vi "UHR-Fleezers Control (host) - 12.8.1.vi"() -> ()   [LabVIEW 2012] (continued)
          tunnel: ["W/ Offset 1"] -> w675
          tunnel: w678 -> [w724]
          tunnel: w675 -> [w722]
          frame #0 {
            n416 = property on="Sample Channel\nFlow" class="Bool (strict)"("Val(Sgnl)"="Daq spot flow on") -> ()  [unwired: 2 in, 2 out]
            n417 = Wait (ms)(milliseconds to wait=u32 250) -> ()  [unwired: 1 out]
          }
          frame #1 {
            n418 = local read "Saved Stage Positions"() -> (w687:dbl[][])
            n419 = property on="Trap Delta (MHz)" class="DigNum (strict)"("Val(Sgnl)"="Cal @ (MHz)") -> ()  [unwired: 2 in, 2 out]
            n420 = local write "Stage Moving"(TRUE ("Stage Moving")) -> ()
            n421 = call "move to saved stage position.vi"("error in"=w689, "Stage VISA resource name in"=w690, "Position"="Cal Stage Position", "Saved Stage Positions"=w687) -> ("error out"=w688:errorcluster)  [unwired: 1 out]
            n422 = local write "Stage Control Serial Error"(w688) -> ()
          }
          frame #2 {
            n423 = local write "Stage Moving"(FALSE ("Stage Moving")) -> ()
            n424 = property on="Sample Channel\nFlow" class="Bool (strict)"("Val(Sgnl)"="Flow ON during cal?") -> ()  [unwired: 2 in, 2 out]
            n425 = call <vilib>:"Beep.vi"() -> ()  [unwired: 3 in, 9 out]
          }
          frame #3 {
            n426 = Wait (ms)(milliseconds to wait=u32 1000) -> ()  [unwired: 1 out]
          }
          frame #4 {
            n427 = property on="Save Calibration" class="Bool (strict)"("Val(Sgnl)"=TRUE ("Value (Signaling)")) -> ()  [unwired: 2 in, 2 out]
          }
          frame #5 {
            n428 = Wait (ms)(milliseconds to wait=u32 2000) -> ()  [unwired: 1 out]
          }
          frame #6 {
            # "Check to see if \nsaving done"
            n429 = while {
              stop <- w699 stop-if-true
              n430 = local read "Saving..."() -> (w700:bool)
              n431 = Wait (ms)(milliseconds to wait=u32 100) -> ()  [unwired: 1 out]
              n432 = Not(x=w700) -> (.not. x?=w699:bool)
            }
          }
          frame #7 {
            n433 = case shown="True" "W/ Offset 1" {
              tunnel: w703 -> [_ w704]
              frame False {
              }
              frame True {
                n434 = stacked-sequence {
                  tunnel: w704 -> [_ _ _ _ _ _ _ w721]
                  frame #0 {
                    n435 = property on="Trap Delta (MHz)" class="DigNum (strict)"("Val(Sgnl)"="Offset 1 Start (MHz)") -> ()  [unwired: 2 in, 2 out]
                    n436 = Replace Array Subset(array=u32[] [0] ("Index Values"), new element="Offset 1 Set", index=0) -> (w705:u32[])
                    n437 = property on="Saved AOD Raster Scan Parameter Sets" class="Arr (strict)"("Index Values"=w705) -> ()  [unwired: 2 in, 2 out]
                  }
                  frame #1 {
                    n438 = Wait (ms)(milliseconds to wait=u32 200) -> ()  [unwired: 1 out]
                  }
                  frame #2 {
                    n439 = property on="Load parameters" class="Bool (strict)"("Val(Sgnl)"=TRUE ("Value (Signaling)")) -> ()  [unwired: 2 in, 2 out]
                  }
                  frame #3 {
                    n440 = Wait (ms)(milliseconds to wait=u32 200) -> ()  [unwired: 1 out]
                  }
                  frame #4 {
                    n441 = property on="Trap Raster Scan" class="Bool (strict)"("Val(Sgnl)"=TRUE ("Value (Signaling)")) -> ()  [unwired: 2 in, 2 out]
                  }
                  frame #5 {
                    n442 = Wait (ms)(milliseconds to wait=u32 2000) -> ()  [unwired: 1 out]
                  }
                  frame #6 {
                    n443 = while {
                      stop <- w718 stop-if-true
                      n444 = local read "Raster Scanning..."() -> (w720:bool)
                      n445 = local read "Saving..."() -> (w716:bool)
                      n446 = Wait (ms)(milliseconds to wait=u32 100) -> ()  [unwired: 1 out]
                      n447 = Not(x=w716) -> (.not. x?=w715:bool)
                      n448 = Not(x=w720) -> (.not. x?=w717:bool)
                      n449 = And(x=w717, y=w715) -> (x .and. y?=w718:bool)
                    }
                  }
                  frame #7 {
                    n450 = property on="Trap Delta (MHz)" class="DigNum (strict)"("Val(Sgnl)"=w721) -> ()  [unwired: 2 in, 2 out]
                  }
                }
              }
            }
          }
          frame #8 {
            n451 = local read "Save ave N"() -> (w723:dbl)
            n452 = case shown="False" "W/ Offset 2" {
              tunnel: w724 -> [_ w731]
              tunnel: w723 -> [_ w730]
              tunnel: w722 -> [w726 _]
              frame False {
                n453 = case shown="False" w726 {
                  frame False {
                    n454 = Multiply(x="Cal read wait (s)", y=u32 1000 ("milliseconds to wait")) -> (x*y=w728:u32)
                    n455 = Wait (ms)(milliseconds to wait=w728) -> ()  [unwired: 1 out]
                  }
                  frame True {
                  }
                }
              }
              frame True {
                n456 = stacked-sequence {
                  tunnel: w731 -> [_ _ _ _ _ _ _ _ _ w752 _ _]
                  tunnel: w730 -> [_ _ _ _ _ _ _ _ _ w750 _ _]
                  frame #0 {
                    n457 = property on="Save ave N" class="DigNum (strict)"("Val(Sgnl)"=1.0 ("Value (Signaling)")) -> ()  [unwired: 2 in, 2 out]
                  }
                  frame #1 {
                    n458 = Wait (ms)(milliseconds to wait=u32 500) -> ()  [unwired: 1 out]
                  }
                  frame #2 {
                    n459 = property on="Trap Delta (MHz)" class="DigNum (strict)"("Val(Sgnl)"="Offset 2 Start (MHz)") -> ()  [unwired: 2 in, 2 out]
                    n460 = Replace Array Subset(array=u32[] [0] ("Index Values"), new element="Offset 2 Set", index=0) -> (w736:u32[])
                    n461 = property on="Saved AOD Raster Scan Parameter Sets" class="Arr (strict)"("Index Values"=w736) -> ()  [unwired: 2 in, 2 out]
                  }
                  frame #3 {
                    n462 = Wait (ms)(milliseconds to wait=u32 500) -> ()  [unwired: 1 out]
                  }
                  frame #4 {
                    n463 = property on="Load parameters" class="Bool (strict)"("Val(Sgnl)"=TRUE ("Value (Signaling)")) -> ()  [unwired: 2 in, 2 out]
                  }
                  frame #5 {
                    n464 = Wait (ms)(milliseconds to wait=u32 500) -> ()  [unwired: 1 out]
                  }
                  frame #6 {
                    n465 = property on="Trap Raster Scan" class="Bool (strict)"("Val(Sgnl)"=TRUE ("Value (Signaling)")) -> ()  [unwired: 2 in, 2 out]
                  }
                  frame #7 {
                    n466 = Wait (ms)(milliseconds to wait=u32 2000) -> ()  [unwired: 1 out]
                  }
                  frame #8 {
                    n467 = while {
                      stop <- w745 stop-if-true
                      n468 = local read "Raster Scanning..."() -> (w748:bool)
                      n469 = local read "Saving..."() -> (w746:bool)
                      n470 = Wait (ms)(milliseconds to wait=u32 100) -> ()  [unwired: 1 out]
                      n471 = Not(x=w746) -> (.not. x?=w744:bool)
                      n472 = Not(x=w748) -> (.not. x?=w747:bool)
                      n473 = And(x=w747, y=w744) -> (x .and. y?=w745:bool)
                    }
                  }
                  frame #9 {
                    n474 = property on="Trap Delta (MHz)" class="DigNum (strict)"("Val(Sgnl)"=w752) -> ()  [unwired: 2 in, 2 out]
                    n475 = property on="Saved AOD Raster Scan Parameter Sets" class="Arr (strict)"("Index Values"=u32[] [0]) -> ()  [unwired: 2 in, 2 out]
                    n476 = property on="Save ave N" class="DigNum (strict)"("Val(Sgnl)"=w750) -> ()  [unwired: 2 in, 2 out]
                  }
                  frame #10 {
                    n477 = Wait (ms)(milliseconds to wait=u32 500) -> ()  [unwired: 1 out]
                  }
                  frame #11 {
                    n478 = property on="Load parameters" class="Bool (strict)"("Val(Sgnl)"=TRUE ("Value (Signaling)")) -> ()  [unwired: 2 in, 2 out]
                  }
                }
              }
            }
          }
          frame #9 {
            n479 = property on="Read Cal" class="Bool (strict)"("Val(Sgnl)"=TRUE ("Value (Signaling)")) -> ()  [unwired: 2 in, 2 out]
          }
          frame #10 {
            n480 = Wait (ms)(milliseconds to wait=u32 1000) -> ()  [unwired: 1 out]
          }
          frame #11 {
            n481 = property on="Fish for Tether" class="Bool (strict)"("Val(Sgnl)"=TRUE ("Value (Signaling)")) -> ()  [unwired: 2 in, 2 out]
          }
        }
        n482 = local write "Cal/Data Acq. Spot"(FALSE ("Cal/Data Acq. Spot")) -> ()
      }
      event "Dump Beads": Value Change {
        n483 = event-data() -> ()  [unwired: 1 in, 5 out]
        n484 = flat-sequence {
          tunnel: ["Dump spot flow on?"] -> w758
          tunnel: [w769] -> w759
          tunnel: w758 -> [w769]
          tunnel: w762 -> [w774]
          tunnel: w761 -> [w773]
          tunnel: [w771] -> w760
          tunnel: w759 -> [w771]
          tunnel: w760 -> [w784]
          frame #0 {
            w763 = FALSE ("Value (Signaling)")
            n485 = local read "Saving..."() -> (w765:bool)
            n486 = local write "Dump Beads"(FALSE ("Dump Beads")) -> ()
            n487 = property on="Inject Pump 3" class="Bool (strict)"("Val(Sgnl)"=w763) -> ()  [unwired: 2 in, 2 out]
            n488 = property on="Inject Pump 1" class="Bool (strict)"("Val(Sgnl)"=w763) -> ()  [unwired: 2 in, 2 out]
            n489 = local write "Stop Saving"(w765) -> ()
          }
          frame #1 {
            w766 = FALSE ("Fl. Triggered...")
            n490 = case shown="True" "Dump spot flow on?" {
              frame False {
              }
              frame True {
                n491 = property on="Sample Channel\nFlow" class="Bool (strict)"("Val(Sgnl)"=TRUE ("Stage Moving")) -> ()  [unwired: 2 in, 2 out]
              }
            }
            n492 = local write "Fl. Triggered..."(w766) -> ()
            n493 = local write "Tether"(w766) -> ()
            n494 = property on="Green Laser ON" class="Bool (strict)"("Val(Sgnl)"=w766) -> ()  [unwired: 2 in, 2 out]
            n495 = property on="Trap Pos. FB ON" class="Bool (strict)"("Val(Sgnl)"=w766) -> ()  [unwired: 2 in, 2 out]
            n496 = property on="Trap Trig. Fl." class="Bool (strict)"("Val(Sgnl)"=w766) -> ()  [unwired: 2 in, 2 out]
            n497 = property on="Fl. Triggered..." class="Bool (strict)"("Val(Sgnl)"=w766) -> ()  [unwired: 2 in, 2 out]
            n498 = property on="Dip for Protein" class="Bool (strict)"("Val(Sgnl)"=w766) -> ()  [unwired: 2 in, 2 out]
            n499 = property on="Pause dwell" class="Bool (strict)"("Val(Sgnl)"=w766) -> ()  [unwired: 2 in, 2 out]
          }
          frame #2 {
            n500 = property on="Trap Pos. FB Offset Factor" class="DigNum (strict)"("Val(Sgnl)"=i64 0 ("Value (Signaling)")) -> ()  [unwired: 2 in, 2 out]
          }
          frame #3 {
            n501 = local read "Saved Stage Positions"() -> (w775:dbl[][])
            n502 = local write "Stage Moving"(TRUE ("Stage Moving")) -> ()
            n503 = Array Subset(array=w775, index (row)=3 ("index"), length (row)=1 ("length"), index (col)=1 ("index"), length (col)=3 ("length")) -> (w780:dbl[][])
            n504 = Reshape Array(w780, 3 ("dimension size")) -> (w778:dbl[])
            n505 = Array To Cluster(array=w778) -> (cluster=w777:cluster{"[0]":dbl, "[1]":dbl, "[2]":dbl})
            n506 = call "Set Stage Position.vi"("Position"=w777, "error in"=w773, "VISA resource name in"=w774) -> ()  [unwired: 3 out]
          }
          frame #4 {
            w785 = FALSE ("Value (Signaling)")
            n507 = case shown="True" w784 {
              frame False {
              }
              frame True {
                n508 = property on="Sample Channel\nFlow" class="Bool (strict)"("Val(Sgnl)"=FALSE ("Stage Moving")) -> ()  [unwired: 2 in, 2 out]
              }
            }
            n509 = property on="Trap 1 (ON/OFF)" class="Bool (strict)"("Val(Sgnl)"=w785) -> ()  [unwired: 2 in, 2 out]
            n510 = property on="Trap 2 (ON/OFF)" class="Bool (strict)"("Val(Sgnl)"=w785) -> ()  [unwired: 2 in, 2 out]
            n511 = call <vilib>:"Beep.vi"() -> ()  [unwired: 3 in, 9 out]
          }
          frame #5 {
            n512 = property on="Move Cap. 2 (ADig Top)" class="Bool (strict)"("Val(Sgnl)"=TRUE ("Value (Signaling)")) -> ()  [unwired: 2 in, 2 out]
            n513 = property on="Tab Control" class="TabCtl (strict)"("Val(Sgnl)"=T30."Status" ("Value (Signaling)")) -> ()  [unwired: 2 in, 2 out]
          }
        }
      }
      event "Dip for Protein": Value Change {
        n514 = event-data() -> ()  [unwired: 1 in, 5 out]
        n515 = case shown="True" "Dip for Protein" {
          tunnel: w791 -> [_ w793]
          tunnel: w790 -> [_ w792]
          frame False {
          }
          frame True {
            n516 = while {
              tunnel: w793 -> [w804]
              tunnel: w792 -> [w803]
              i -> [w798]
              stop <- w800 stop-if-true
              n517 = Increment(x=w798) -> (x+1=→"Dip #":i32)
              n518 = flat-sequence {
                tunnel: w803 -> [w815]
                tunnel: w804 -> [w816]
                tunnel: [w816] -> w808
                tunnel: [w815] -> w807
                tunnel: [w809] -> w794
                tunnel: [w821] -> w802
                tunnel: [w822] -> w801
                tunnel: w808 -> [w823]
                tunnel: w807 -> [w824]
                tunnel: [w819] -> w795
                tunnel: w794 -> [w819]
                tunnel: [w832] -> w806
                tunnel: w802 -> [w832]
                tunnel: [w831] -> w805
                tunnel: w801 -> [w831]
                tunnel: [w828] -> w799
                tunnel: [w827] -> w796
                tunnel: w795 -> [w827]
                tunnel: w805 -> [w852]
                tunnel: w806 -> [w853]
                tunnel: w799 -> [w854]
                tunnel: w796 -> [w851]
                tunnel: [w910] -> w800
                frame #0 {
                  n519 = local read "Trap Pos. FB ON"() -> (w809:bool)
                  n520 = Compound Arithmetic op=AND("Flow ON\nduring dip?", "FB OFF when \nflow ON", w809) -> (w810:bool)
                  n521 = case shown="True" "Move trap \nbefore dip move?" {
                    frame False {
                    }
                    frame True {
                      n522 = property on="Trap Delta (MHz)" class="DigNum (strict)"("Val(Sgnl)"="Dipping Delta (MHz)") -> ()  [unwired: 2 in, 2 out]
                    }
                  }
                  n523 = property on="Green Laser ON" class="Bool (strict)"("Val(Sgnl)"="Green ON\nbefore dip?") -> ()  [unwired: 2 in, 2 out]
                  n524 = property on="Sample Channel\nFlow" class="Bool (strict)"("Val(Sgnl)"="Flow ON\nduring dip?") -> ()  [unwired: 2 in, 2 out]
                  n525 = case shown="True" w810 {
                    frame False {
                    }
                    frame True {
                      n526 = property on="Trap Pos. FB ON" class="Bool (strict)"("Val(Sgnl)"=FALSE ("Value (Signaling)")) -> ()  [unwired: 2 in, 2 out]
                    }
                  }
                }
                frame #1 {
                  n527 = local read "Saved Stage Positions"() -> (w826:dbl[][])
                  n528 = local write "Cancel dwell"(FALSE ("Cancel dwell")) -> ()
                  n529 = call "move to saved stage position.vi"("error in"=w824, "Stage VISA resource name in"=w823, "Position"="Dip Stage \nPosition", "Saved Stage Positions"=w826) -> ("VISA resource name out"=w821:refnum<visa-resource-name>, "error out"=w822:errorcluster)
                }
                frame #2 {
                  n530 = node-c288() -> (w830:T27)  [unwired: 4 in]
                  n531 = timed-loop {
                    timing: w830 -> [_]
                    timing-out: [_] -> w829
                    tunnel: [w836] -> w828
                    i -> [w833]
                    stop <- w837 stop-if-true
                    n532 = node-c288() -> ()  [unwired: 1 in, 1 out]
                    n533 = Greater Or Equal?(x=w833, y="Dip Duration (s)") -> (x >= y?=w845:bool)
                    n534 = local read "Dip for Protein"() -> (w838:bool)
                    n535 = local read "Dump Beads"() -> (w835:bool)
                    n536 = local read "Cancel dwell"() -> (w844:bool)
                    n537 = local read "Pause dwell"() -> (w841:bool)
                    n538 = Not(x=w838) -> (.not. x?=w843:bool)
                    n539 = Compound Arithmetic op=OR(w844, w845, w843) -> (w842:bool)
                    n540 = Select(t=FALSE, s=w841, f=w842) -> (s? t:f=w839:bool)
                    n541 = Not(x=w835) -> (.not. x?=w834:bool)
                    n542 = node-c288() -> ()  [unwired: 1 in, 1 out]
                    n543 = And(x=w838, y=w834) -> (x .and. y?=w836:bool)
                    n544 = Or(x=w839, y=w835) -> (x .or. y?=w837:bool)
                    "Dip Time (s)" <- w833
                  }
                  n545 = node-c288(w829) -> ()  [unwired: 1 out]
                }
                frame #3 {
                  n546 = case shown="True" w854 {
                    tunnel: w853 -> [_ w859]
                    tunnel: w852 -> [_ w858]
                    tunnel: w851 -> [_ w855]
                    frame False {
                    }
                    frame True {
                      n547 = flat-sequence {
                        tunnel: w858 -> [w863]
                        tunnel: w859 -> [w864]
                        tunnel: [w864] -> w857
                        tunnel: [w863] -> w856
                        tunnel: w855 -> [w860]
                        tunnel: w857 -> [w874]
                        tunnel: w856 -> [w873]
                        tunnel: w855 -> [w882]
                        frame #0 {
                          n548 = local read "Sample Channel\nFlow"() -> (w862:bool)
                          n549 = case shown="True" w862 {
                            tunnel: "Flow ON \nduring return\nfrom dip?" -> [w865 w868]
                            tunnel: w860 -> [_ w867]
                            frame False {
                              n550 = case shown="True" w865 {
                                frame False {
                                }
                                frame True {
                                n551 = property on="Sample Channel\nFlow" class="Bool (strict)"("Val(Sgnl)"=TRUE ("Value (Signaling)")) -> ()  [unwired: 2 in, 2 out]
                                }
                              }
                            }
                            frame True {
                              n552 = case shown="False" w868 {
                                tunnel: w867 -> [w869 _]
                                frame False {
                                n553 = property on="Trap Pos. FB ON" class="Bool (strict)"("Val(Sgnl)"=w869) -> ()  [unwired: 2 in, 2 out]
                                n554 = property on="Sample Channel\nFlow" class="Bool (strict)"("Val(Sgnl)"=FALSE ("Value (Signaling)")) -> ()  [unwired: 2 in, 2 out]
                                }
                                frame True {
                                }
                              }
                            }
                          }
                        }
                        frame #1 {
                          # "For turning on green laser before stage reaches lower spot"
                          n555 = case shown="True" "Green ON\nafter start\nreturn?" {
                            frame False {
                            }
                            frame True {
                              n556 = flat-sequence {
                                frame #0 {
                                n557 = Multiply(x="Green delay after \nstart return (s)", y=1000.0) -> (x*y=w879:dbl)
                                n558 = Wait (ms)(milliseconds to wait=w879) -> ()  [unwired: 1 out]
                                }
                                frame #1 {
                                n559 = property on="Green Laser ON" class="Bool (strict)"("Val(Sgnl)"=TRUE ("Value (Signaling)")) -> ()  [unwired: 2 in, 2 out]
                                }
                              }
                            }
                          }
                          n560 = local read "Saved Stage Positions"() -> (w877:dbl[][])
                          n561 = local write "Cancel dwell"(FALSE ("Cancel dwell")) -> ()
                          n562 = call "move to saved stage position.vi"("error in"=w873, "Stage VISA resource name in"=w874, "Position"="Return Stage \nPosition", "Saved Stage Positions"=w877) -> ("error out"=w875:errorcluster)  [unwired: 1 out]
                          n563 = local write "Stage Control Serial Error"(w875) -> ()
                        }
                        frame #2 {
                          n564 = property on="Trap Pos. FB ON" class="Bool (strict)"("Val(Sgnl)"=w882) -> ()  [unwired: 2 in, 2 out]
                          n565 = case shown="True" "Green ON \nafter return?" {
                            frame False {
                            }
                            frame True {
                              n566 = property on="Green Laser ON" class="Bool (strict)"("Val(Sgnl)"=TRUE ("Value (Signaling)")) -> ()  [unwired: 2 in, 2 out]
                            }
                          }
                          n567 = case shown="True" "Move trap after return?" {
                            frame False {
                            }
                            frame True {
                              n568 = property on="Trap Delta (MHz)" class="DigNum (strict)"("Val(Sgnl)"="Dip Trap Delta 2 (MHz)") -> ()  [unwired: 2 in, 2 out]
                            }
                          }
                          n569 = case shown="True" "Save data after return?" {
                            frame False {
                            }
                            frame True {
                              n570 = property on="Start Saving" class="Bool (strict)"("Val(Sgnl)"=TRUE ("Value (Signaling)")) -> ()  [unwired: 2 in, 2 out]
                            }
                          }
                          n571 = property on="Sample Channel\nFlow" class="Bool (strict)"("Val(Sgnl)"="Flow ON\nduring daq?") -> ()  [unwired: 2 in, 2 out]
                        }
                        frame #3 {
                          n572 = node-c288() -> (w891:T27)  [unwired: 4 in]
                          n573 = timed-loop {
                            timing: w891 -> [_]
                            timing-out: [_] -> w890
                            i -> [w892]
                            stop <- w894 stop-if-true
                            n574 = node-c288() -> ()  [unwired: 1 in, 1 out]
                            n575 = local read "Dump Beads"() -> (w893:bool)
                            n576 = Greater Or Equal?(x=w892, y="Dwell Duration (s)") -> (x >= y?=w899:bool)
                            n577 = local read "Dip for Protein"() -> (w896:bool)
                            n578 = Not(x=w896) -> (.not. x?=w895:bool)
                            n579 = Compound Arithmetic op=OR(w899, "Cancel dwell", w895) -> (w898:bool)
                            n580 = node-c288() -> ()  [unwired: 1 in, 1 out]
                            n581 = Select(t=FALSE, s="Pause dwell", f=w898) -> (s? t:f=w901:bool)
                            n582 = Or(x=w901, y=w893) -> (x .or. y?=w894:bool)
                            "Dwell Time (s)" <- w892
                          }
                          n583 = node-c288(w890) -> ()  [unwired: 1 out]
                        }
                      }
                    }
                  }
                }
                frame #4 {
                  n584 = local read "Dip for Protein"() -> (w911:bool)
                  n585 = local read "Dump Beads"() -> (w908:bool)
                  n586 = local write "Cancel dwell"(FALSE ("Cancel dwell")) -> ()
                  n587 = Not(x=w911) -> (.not. x?=w912:bool)
                  n588 = Not(x="Cont. Repeat Dipping?") -> (.not. x?=w914:bool)
                  n589 = Compound Arithmetic op=OR(w912, w914, w908) -> (w910:bool)
                }
              }
            }
          }
        }
      }
      event "Profile": Value Change {
        n590 = event-data() -> ()  [unwired: 1 in, 5 out]
        n591 = flat-sequence {
          tunnel: w923 -> [w926]
          tunnel: w922 -> [w934]
          tunnel: [w928] -> w921
          tunnel: [w927] -> w920
          tunnel: [w925] -> w918
          tunnel: [w924] -> w915
          tunnel: w921 -> [w941]
          tunnel: w920 -> [w940]
          tunnel: [w938] -> w919
          tunnel: w918 -> [w939]
          tunnel: [w937] -> w917
          tunnel: [w936] -> w916
          tunnel: w915 -> [w936]
          tunnel: w919 -> [w945]
          tunnel: w917 -> [w944]
          tunnel: w916 -> [w943]
          frame #0 {
            n592 = call "Read Stage Position.vi"("error in"=w934, "VISA resource name in"=w926) -> ("Current Position"=w924:cluster{dbl, dbl, dbl}, "error out"=w927:errorcluster, "VISA resource name out"=w925:refnum<visa-resource-name>)  [unwired: 1 out]
            "Current Position" <- w924
            n593 = local write "Stage Control Serial Error"(w927) -> ()
            n594 = Unbundle(w924) -> (w931:dbl, w933:dbl, w929:dbl)
            n595 = Add(x=w933, y="Y change (mm)") -> (x+y=w930:dbl)
            n596 = Bundle(w931, w930, w929) -> (w928:cluster{dbl, dbl, dbl})  [unwired: 1 in]
          }
          frame #1 {
            # "move to new position and start saving"
            n597 = local write "Stage Moving"(TRUE ("Stage Moving")) -> ()
            n598 = local write "Start Saving"(TRUE ("Start Saving")) -> ()
            n599 = call "Set Stage Position.vi"("Position"=w941, "error in"=w940, "VISA resource name in"=w939) -> ("error out"=w937:errorcluster, "VISA resource name out"=w938:refnum<visa-resource-name>)  [unwired: 1 out]
          }
          frame #2 {
            # "go back to start"
            n600 = call "Set Stage Position.vi"("Position"=w943, "error in"=w944, "VISA resource name in"=w945) -> ()  [unwired: 3 out]
          }
          frame #3 {
            # "stop saving"
            n601 = local write "Stop Saving"(TRUE ("Stop Saving")) -> ()
            n602 = local write "Stage Moving"(FALSE ("Stage Moving")) -> ()
          }
        }
      }
      event "Move to Position 1", "Move to Position 2", "Move to Position 3", "Move to Position 4", "Move to Position 5", "Lower Ch. Cap.": Value Change {
        n603 = event-data() -> ()  [unwired: 1 in, 5 out]
        n604 = Or(x="Move to Position 5", y="Lower Ch. Cap.") -> (x .or. y?=w951:bool)
        n605 = Build Array("Move to Position 1", "Move to Position 2", "Move to Position 3", "Move to Position 4", w951) -> (w954:bool[])
        n606 = Boolean Array To Number(Boolean array=w954) -> (number=w953:u32)
        n607 = Logarithm Base 2(1:w953) -> (0:w952:dbl)
        n608 = flat-sequence {
          tunnel: w952 -> [w963]
          tunnel: w949 -> [w961]
          tunnel: w948 -> [w960]
          frame #0 {
            n609 = local read "Saved Stage Positions"() -> (w971:dbl[][])
            n610 = Array Subset(array=w971, index (row)=w963, length (row)=1 ("length"), index (col)=1 ("index"), length (col)=3 ("length")) -> (w968:dbl[][])
            n611 = Reshape Array(w968, 3 ("dimension size")) -> (w966:dbl[])
            n612 = Array To Cluster(array=w966) -> (cluster=w965:cluster{"[0]":dbl, "[1]":dbl, "[2]":dbl})
            n613 = call "Set Stage Position.vi"("Position"=w965, "error in"=w960, "VISA resource name in"=w961) -> ("error out"=w964:errorcluster)  [unwired: 2 out]
            n614 = local write "Stage Moving"(TRUE ("Stage Moving")) -> ()
            n615 = local write "Stage Control Serial Error"(w964) -> ()
          }
          frame #1 {
            n616 = local write "Stage Moving"(FALSE ("Stage Moving")) -> ()
            n617 = call <vilib>:"Beep.vi"() -> ()  [unwired: 3 in, 9 out]
          }
        }
      }
      event "Got ADig bead": Value Change {
        n618 = event-data() -> ()  [unwired: 1 in, 5 out]
        n619 = flat-sequence {
          frame #0 {
            n620 = local read "Cap 1 Samp Flow ON"() -> (w975:bool)
            n621 = case shown="True" w975 {
              frame False {
              }
              frame True {
                n622 = property on="Sample Channel\nFlow" class="Bool (strict)"("Val(Sgnl)"=TRUE ("Value (Signaling)")) -> ()  [unwired: 2 in, 2 out]
              }
            }
          }
          frame #1 {
            n623 = property on="Inject Pump 3" class="Bool (strict)"("Val(Sgnl)"=FALSE ("Value (Signaling)")) -> ()  [unwired: 2 in, 2 out]
          }
          frame #2 {
            n624 = property on="Move Cap. 1 (DNA Bottom)" class="Bool (strict)"("Val(Sgnl)"=TRUE ("Value (Signaling)")) -> ()  [unwired: 2 in, 2 out]
          }
        }
      }
      event "Force FB Data\nScript": Value Change {
        n625 = event-data() -> ()  [unwired: 1 in, 5 out]
        n626 = flat-sequence {
          tunnel: w984 -> [w988]
          tunnel: w985 -> [w989]
          tunnel: [w989] -> w980
          tunnel: [w988] -> w979
          tunnel: w980 -> [w992]
          tunnel: w979 -> [w991]
          tunnel: ["Trap Trig Fl."] -> w981
          tunnel: [w1017] -> w982
          tunnel: w981 -> [w1017]
          tunnel: [w1021] -> w983
          tunnel: w982 -> [w1021]
          tunnel: w983 -> [w1023]
          frame #0 {
            n627 = property on="Trap Delta (MHz)" class="DigNum (strict)"("Val(Sgnl)"="Trap Delta Before Moving") -> ()  [unwired: 2 in, 2 out]
          }
          frame #1 {
            n628 = local read "Saved Stage Positions"() -> (w994:dbl[][])
            n629 = local write "FB Trap Pos Offset"(0.0 ("FB Trap Pos Offset")) -> ()
            n630 = property on="Trap Pos. FB Offset Factor" class="DigNum (strict)"("Val(Sgnl)"=i64 0 ("Value (Signaling)")) -> ()  [unwired: 2 in, 2 out]
            n631 = local write "Stage Moving"(TRUE ("Stage Moving")) -> ()
            n632 = call "move to saved stage position.vi"("error in"=w991, "Stage VISA resource name in"=w992, "Position"="Stage Position To Establish FB", "Saved Stage Positions"=w994) -> ("error out"=w990:errorcluster)  [unwired: 1 out]
            n633 = local write "Stage Control Serial Error"(w990) -> ()
          }
          frame #2 {
            n634 = call <vilib>:"Beep.vi"() -> ()  [unwired: 3 in, 9 out]
            n635 = Multiply(x="Wait (s)", y=u32 1000 ("milliseconds to wait")) -> (x*y=w1001:u32)
            n636 = property on="Trap Delta (MHz)" class="DigNum (strict)"("Val(Sgnl)"="Starting \nTrap Delta (MHz)") -> ()  [unwired: 2 in, 2 out]
            n637 = local write "Stage Moving"(FALSE ("Stage Moving")) -> ()
            n638 = Wait (ms)(milliseconds to wait=w1001) -> ()  [unwired: 1 out]
            n639 = property on="Tab Control 2" class="TabCtl (strict)"("Val(Sgnl)"=T8."Feedback on Trap Position" ("Value (Signaling)")) -> ()  [unwired: 2 in, 2 out]
            n640 = property on="Tab Control" class="TabCtl (strict)"("Val(Sgnl)"=T31."Trap Control (RF)" ("Value (Signaling)")) -> ()  [unwired: 2 in, 2 out]
          }
          frame #3 {
            n641 = property on="Set Reading to\nSetpoint" class="Bool (strict)"("Val(Sgnl)"=TRUE ("Value (Signaling)")) -> ()  [unwired: 2 in, 2 out]
            n642 = Wait (ms)(milliseconds to wait=u32 500) -> ()  [unwired: 1 out]
          }
          frame #4 {
            n643 = property on="Trap Pos. FB ON" class="Bool (strict)"("Val(Sgnl)"=TRUE ("Value (Signaling)")) -> ()  [unwired: 2 in, 2 out]
            n644 = Wait (ms)(milliseconds to wait=u32 250) -> ()  [unwired: 1 out]
          }
          frame #5 {
            n645 = case shown="False" "Trap Trig Fl." {
              frame False {
                n646 = case shown="True" "Green ON after FB ON?" {
                  selector: "Green ON after FB ON?" -> [_ w1016]
                  frame False {
                  }
                  frame True {
                    n647 = property on="Green Laser ON" class="Bool (strict)"("Val(Sgnl)"=w1016) -> ()  [unwired: 2 in, 2 out]
                  }
                }
              }
              frame True {
              }
            }
            n648 = case shown="True" "Remove Action Offset" {
              tunnel: TRUE ("Value (Signaling)") -> [w1013 w1014]
              frame False {
                n649 = property on="Remove Unwinding Offset" class="Bool (strict)"("Val(Sgnl)"=w1013) -> ()  [unwired: 2 in, 2 out]
              }
              frame True {
                n650 = property on="Remove Action Offset" class="Bool (strict)"("Val(Sgnl)"=w1014) -> ()  [unwired: 2 in, 2 out]
              }
            }
            n651 = Wait (ms)(milliseconds to wait=u32 250) -> ()  [unwired: 1 out]
          }
          frame #6 {
            n652 = property on="Start Saving" class="Bool (strict)"("Val(Sgnl)"=TRUE ("Value (Signaling)")) -> ()  [unwired: 2 in, 2 out]
            n653 = Wait (ms)(milliseconds to wait=u32 5000) -> ()  [unwired: 1 out]
          }
          frame #7 {
            w1020 = TRUE ("Value (Signaling)")
            n654 = property on="Rem fb disp offset" class="Bool (strict)"("Val(Sgnl)"=w1020) -> ()  [unwired: 2 in, 2 out]
            n655 = property on="Remove Offset" class="Bool (strict)"("Val(Sgnl)"=w1020) -> ()  [unwired: 2 in, 2 out]
            n656 = Wait (ms)(milliseconds to wait=u32 100) -> ()  [unwired: 1 out]
          }
          frame #8 {
            n657 = case shown="True" w1023 {
              frame False {
              }
              frame True {
                n658 = local write "Trap Trig. Fl."(TRUE ("Value (Signaling)")) -> ()
              }
            }
          }
          frame #9 {
            n659 = case shown="True" "Start dipping after?" {
              frame False {
              }
              frame True {
                n660 = flat-sequence {
                  frame #0 {
                    n661 = Multiply(x="Delay before dipping (s)", y=1000.0) -> (x*y=w1027:dbl)
                    n662 = Wait (ms)(milliseconds to wait=w1027) -> ()  [unwired: 1 out]
                  }
                  frame #1 {
                    n663 = property on="Dip for Protein" class="Bool (strict)"("Val(Sgnl)"=TRUE ("Value (Signaling)")) -> ()  [unwired: 2 in, 2 out]
                    n664 = local write "Scripts"(T1."Dipping" ("Scripts")) -> ()
                  }
                }
              }
            }
          }
        }
      }
      event "Fixed Traps Data\nScript": Value Change {
        n665 = event-data() -> ()  [unwired: 1 in, 5 out]
        n666 = flat-sequence {
          frame #0 {
            n667 = case shown="True" "Green ON" {
              frame False {
              }
              frame True {
                n668 = property on="Green Laser ON" class="Bool (strict)"("Val(Sgnl)"=TRUE) -> ()  [unwired: 2 in, 2 out]
              }
            }
            n669 = local write "Offset (nm)"(0.0 ("Offset (nm)")) -> ()
            n670 = property on="Sample Channel\nFlow" class="Bool (strict)"("Val(Sgnl)"=FALSE ("Value (Signaling)")) -> ()  [unwired: 2 in, 2 out]
            n671 = property on="Trap Delta (MHz)" class="DigNum (strict)"("Val(Sgnl)"="Fixed Traps Trap Delta (MHz)") -> ()  [unwired: 2 in, 2 out]
          }
          frame #1 {
            n672 = Wait (ms)(milliseconds to wait=u32 1000) -> ()  [unwired: 1 out]
          }
          frame #2 {
            n673 = local write "Start Saving"(TRUE ("Start Saving")) -> ()
          }
          frame #3 {
            n674 = local read "Bead Sep. Int. Time (s)"() -> (w1038:dbl)
            n675 = Multiply(x=w1038, y=1000.0) -> (x*y=w1040:dbl)
            n676 = Wait (ms)(milliseconds to wait=w1040) -> ()  [unwired: 1 out]
          }
          frame #4 {
            n677 = property on="Remove Offset" class="Bool (strict)"("Val(Sgnl)"=TRUE ("Value (Signaling)")) -> ()  [unwired: 2 in, 2 out]
          }
          frame #5 {
            n678 = property on="Dip for Protein" class="Bool (strict)"("Val(Sgnl)"="Start dipping after?") -> ()  [unwired: 2 in, 2 out]
          }
        }
      }
      event "Got DNA bead": Value Change {
        n679 = event-data() -> ()  [unwired: 1 in, 5 out]
        n680 = flat-sequence {
          frame #0 {
            n681 = local read "Daq spot flow on"() -> (w1045:bool)
            n682 = case shown="True" w1045 {
              frame False {
              }
              frame True {
                n683 = property on="Sample Channel\nFlow" class="Bool (strict)"("Val(Sgnl)"=TRUE ("Value (Signaling)")) -> ()  [unwired: 2 in, 2 out]
              }
            }
            n684 = property on="Got DNA bead" class="Bool"("Key Focus"=FALSE) -> ()  [unwired: 2 in, 2 out]
          }
          frame #1 {
            n685 = property on="Inject Pump 1" class="Bool (strict)"("Val(Sgnl)"=FALSE ("Value (Signaling)")) -> ()  [unwired: 2 in, 2 out]
          }
          frame #2 {
            n686 = property on="Cal/Data Acq. Spot" class="Bool (strict)"("Val(Sgnl)"=TRUE ("Value (Signaling)")) -> ()  [unwired: 2 in, 2 out]
          }
        }
      }
      event "Take Stepping Data": Value Change {
        n687 = event-data() -> ()  [unwired: 1 in, 5 out]
        n688 = local read "Save ave N"() -> (w1057:dbl)
        n689 = flat-sequence {
          tunnel: w1057 -> [w1059]
          tunnel: [w1059] -> w1052
          tunnel: [w1061] -> w1053
          tunnel: w1052 -> [w1061]
          tunnel: [w1063] -> w1054
          tunnel: w1053 -> [w1063]
          tunnel: [w1066] -> w1055
          tunnel: w1054 -> [w1066]
          tunnel: [w1068] -> w1056
          tunnel: w1055 -> [w1068]
          tunnel: [w1070] -> w1050
          tunnel: w1056 -> [w1070]
          tunnel: w1050 -> [w1073]
          tunnel: [w1073] -> w1049
          tunnel: w1049 -> [w1074]
          tunnel: [w1074] -> w1051
          tunnel: w1051 -> [w1080]
          frame #0 {
            n690 = property on="Save ave N" class="DigNum (strict)"("Val(Sgnl)"="Save ave factor") -> ()  [unwired: 2 in, 2 out]
          }
          frame #1 {
            n691 = Wait (ms)(milliseconds to wait=u32 100) -> ()  [unwired: 1 out]
          }
          frame #2 {
            n692 = local read "Offset 2 Start (MHz)"() -> (w1065:dbl)
            n693 = property on="Saved AOD Raster Scan Parameter Sets" class="Arr (strict)"("Index Values"=u32[] [2]) -> ()  [unwired: 2 in, 2 out]
            n694 = property on="Trap Delta (MHz)" class="DigNum (strict)"("Val(Sgnl)"=w1065) -> ()  [unwired: 2 in, 2 out]
          }
          frame #3 {
            n695 = property on="Load parameters" class="Bool (strict)"("Val(Sgnl)"=TRUE ("Value (Signaling)")) -> ()  [unwired: 2 in, 2 out]
          }
          frame #4 {
            n696 = Wait (ms)(milliseconds to wait=u32 100) -> ()  [unwired: 1 out]
          }
          frame #5 {
            n697 = property on="Trap Raster Scan" class="Bool (strict)"("Val(Sgnl)"=TRUE ("Value (Signaling)")) -> ()  [unwired: 2 in, 2 out]
          }
          frame #6 {
            n698 = Wait (ms)(milliseconds to wait=u32 1000) -> ()  [unwired: 1 out]
          }
          frame #7 {
            n699 = while {
              stop <- w1077 stop-if-true
              n700 = local read "Raster Scanning..."() -> (w1079:bool)
              n701 = local read "Saving..."() -> (w1078:bool)
              n702 = Not(x=w1078) -> (.not. x?=w1075:bool)
              n703 = Not(x=w1079) -> (.not. x?=w1076:bool)
              n704 = And(x=w1076, y=w1075) -> (x .and. y?=w1077:bool)
            }
          }
          frame #8 {
            n705 = property on="Save ave N" class="DigNum (strict)"("Val(Sgnl)"=w1080) -> ()  [unwired: 2 in, 2 out]
          }
        }
      }
      event "Step Size (nm)": Value Change {
        n706 = event-data() -> ()  [unwired: 1 in, 5 out]
        n707 = flat-sequence {
          frame #0 {
            n708 = property on="Saved AOD Raster Scan Parameter Sets" class="Arr (strict)"("Index Values"=u32[] [1]) -> ()  [unwired: 2 in, 2 out]
          }
          frame #1 {
            n709 = Multiply(x="N Steps", y="Step Size (nm)") -> (x*y=w1082:dbl)
            n710 = property on="Scan Speed AOD (nm/s) 2" class="DigNum (strict)"("Value"="Step Size (nm)") -> ()  [unwired: 2 in, 2 out]
            n711 = property on="Step Size AOD (nm) 2" class="DigNum (strict)"("Value"="Step Size (nm)") -> ()  [unwired: 2 in, 2 out]
            n712 = property on="Scan Range AOD (nm) 2" class="DigNum (strict)"("Value"=w1082) -> ()  [unwired: 2 in, 2 out]
          }
        }
      }
      event "Take Detection Laser\nImage": Value Change {
        n713 = event-data() -> ()  [unwired: 1 in, 5 out]
        n714 = flat-sequence {
          tunnel: [w1110] -> w1100
          tunnel: [w1109] -> w1093
          tunnel: [w1108] -> w1085
          tunnel: [w1113] -> w1101
          tunnel: w1100 -> [w1113]
          tunnel: [w1112] -> w1094
          tunnel: w1093 -> [w1112]
          tunnel: [w1111] -> w1086
          tunnel: w1085 -> [w1111]
          tunnel: [w1117] -> w1102
          tunnel: w1101 -> [w1117]
          tunnel: [w1116] -> w1095
          tunnel: w1094 -> [w1116]
          tunnel: [w1115] -> w1087
          tunnel: w1086 -> [w1115]
          tunnel: [w1123] -> w1103
          tunnel: w1102 -> [w1123]
          tunnel: [w1122] -> w1096
          tunnel: w1095 -> [w1122]
          tunnel: [w1121] -> w1088
          tunnel: w1087 -> [w1121]
          tunnel: [w1127] -> w1104
          tunnel: w1103 -> [w1127]
          tunnel: [w1126] -> w1097
          tunnel: w1096 -> [w1126]
          tunnel: [w1125] -> w1089
          tunnel: w1088 -> [w1125]
          tunnel: [w1131] -> w1105
          tunnel: w1104 -> [w1131]
          tunnel: [w1130] -> w1098
          tunnel: w1097 -> [w1130]
          tunnel: [w1129] -> w1090
          tunnel: w1089 -> [w1129]
          tunnel: [w1135] -> w1106
          tunnel: w1105 -> [w1135]
          tunnel: [w1134] -> w1099
          tunnel: w1098 -> [w1134]
          tunnel: [w1133] -> w1091
          tunnel: w1090 -> [w1133]
          tunnel: w1106 -> [w1141]
          tunnel: w1099 -> [w1140]
          tunnel: [w1138] -> w1092
          tunnel: w1091 -> [w1138]
          tunnel: w1092 -> [w1142]
          frame #0 {
            n715 = local read "Laser interlacing mode"() -> (w1109:enum32{"Laser ON", "Laser OFF", "Interlace"})
            n716 = local read "Green FB On/Off"() -> (w1108:bool)
            n717 = local read "Green Laser ON"() -> (w1110:bool)
          }
          frame #1 {
            n718 = property on="Green FB On/Off" class="Bool (strict)"("Val(Sgnl)"=FALSE ("Value (Signaling)")) -> ()  [unwired: 2 in, 2 out]
          }
          frame #2 {
            n719 = property on="Green Laser ON" class="Bool (strict)"("Val(Sgnl)"=TRUE ("Value (Signaling)")) -> ()  [unwired: 2 in, 2 out]
            n720 = property on="Flip Green Filter" class="Bool (strict)"("Val(Sgnl)"=TRUE ("Value (Signaling)")) -> ()  [unwired: 2 in, 2 out]
            n721 = property on="Laser interlacing mode" class="RadioBtnsControl (strict)"("Val(Sgnl)"=enum32{"Laser ON", "Laser OFF", "Interlace"}."Laser ON" ("Value (Signaling)")) -> ()  [unwired: 2 in, 2 out]
          }
          frame #3 {
            n722 = Wait (ms)(milliseconds to wait=u32 500) -> ()  [unwired: 1 out]
          }
          frame #4 {
            n723 = property on="Confocal Image" class="Bool (strict)"("Val(Sgnl)"=TRUE ("Value (Signaling)")) -> ()  [unwired: 2 in, 2 out]
          }
          frame #5 {
            n724 = Wait (ms)(milliseconds to wait=u32 2000) -> ()  [unwired: 1 out]
          }
          frame #6 {
            n725 = while {
              stop <- w1136 stop-if-true
              n726 = local read "Saving..."() -> (w1137:bool)
              n727 = Not(x=w1137) -> (.not. x?=w1136:bool)
            }
          }
          frame #7 {
            n728 = property on="Flip Green Filter" class="Bool (strict)"("Val(Sgnl)"=TRUE ("Value (Signaling)")) -> ()  [unwired: 2 in, 2 out]
            n729 = property on="Green Laser ON" class="Bool (strict)"("Val(Sgnl)"=w1141) -> ()  [unwired: 2 in, 2 out]
            n730 = property on="Laser interlacing mode" class="RadioBtnsControl (strict)"("Val(Sgnl)"=w1140) -> ()  [unwired: 2 in, 2 out]
          }
          frame #8 {
            n731 = property on="Green FB On/Off" class="Bool (strict)"("Val(Sgnl)"=w1142) -> ()  [unwired: 2 in, 2 out]
          }
        }
      }
      event "Move in a Circle": Value Change {
        w1144 = dbl[] []
        # "converting distance (d) to angle (a)\na=arcsin(d/2r)"
        # "radius"
        # "radius"
        # "T1 Y"
        # "T1 X"
        n732 = event-data() -> ()  [unwired: 1 in, 5 out]
        n733 = local read "BD 1 Frequency 1 (MHz)"() -> (w1152:dbl)
        n734 = local read "BD 2 Frequency 1 (MHz)"() -> (w1151:dbl)
        n735 = local read "BD 1 Frequency 2 (MHz)"() -> (w1150:dbl)
        n736 = local read "BD 2 Frequency 2 (MHz)"() -> (w1149:dbl)
        n737 = Subtract(x=w1151, y="Center Y Frequency (MHz)") -> (x-y=w1156:dbl)
        n738 = Absolute Value(x=w1156) -> (abs(x)=w1147:dbl)
        n739 = flat-sequence {
          tunnel: w1147 -> [w1159]
          tunnel: [w1159] -> w1146
          frame #0 {
            n740 = local write "Radius (MHz)"(w1159) -> ()
          }
        }
        n741 = node-c288("Time step (ms)") -> (w1158:T27)  [unwired: 3 in]
        n742 = timed-loop {
          timing: w1158 -> [_]
          timing-out: [_] -> w1157
          tunnel: w1152 -> [w1250]
          tunnel: w1151 -> [_]
          tunnel: w1150 -> [w1254]
          tunnel: w1149 -> [_]
          tunnel: "Center Y Frequency (MHz)" -> [w1243]
          shift-right: [w1204] -> _
          shift-left: w1144 -> [w1211]
          shift-right: [w1202] -> _
          shift-left: w1144 -> [w1210]
          shift-right: [w1195] -> _
          shift-left: w1144 -> [w1208]
          shift-right: [w1193] -> _
          shift-left: w1144 -> [w1207]
          tunnel: "Move in a Circle" -> [_]
          tunnel: ["Back to start on finish?"] -> w1148
          tunnel: w1146 -> [_]
          tunnel: w1145 -> [w1225]
          tunnel: w1144 -> [w1206]
          shift-right: [w1177] -> _
          shift-left: 0.0 -> [w1175]
          i -> [w1184]
          stop <- w1248 stop-if-true
          w1192 = 0 ("index")
          w1213 = 1 ("dimension size")
          # "Keep phase within\n2pi so errors don't \nbuild"
          # "Accumulated\nphase"
          # "Current phase"
          # "Trap 2"
          # "Trap 1"
          # "ignore if N = 0"
          # "r"
          # "r"
          # "r"
          # "r"
          # "\"omega*t\""
          # "Trap 2"
          # "Trap separation (radians)"
          # "Trap 1"
          # "Offset (starts\n at bottom of\n the circle)"
          # "omega"
          n743 = node-c288() -> (w1261:i64)  [unwired: 1 in]
          n744 = Divide(x=w1261, y=1000) -> (x/y=w1180:dbl)
          n745 = Divide(x="2D Motion Trap Separation (MHz)", y="Radius (MHz)") -> (x/y=w1235:dbl)
          n746 = Negate(x=w1180) -> (-x=w1179:dbl)
          n747 = Divide(x="Trap 2 phase shift (deg)", y=360.0) -> (x/y=w1226:dbl)
          n748 = Inverse Sine(1:w1235) -> (0:w1171:dbl)
          n749 = Multiply(x=6.283185307179586, y=w1226) -> (x*y=w1172:dbl)
          n750 = Multiply(x=6.283185307179586, y="2D Motion Frequency (Hz)") -> (x*y=w1183:dbl)
          n751 = Select(t=w1180, s="Counterclockwise/Clockwise", f=w1179) -> (s? t:f=w1182:dbl)
          n752 = Multiply(x=w1183, y=w1182) -> (x*y=w1173:dbl)
          n753 = Select(t=w1171, s="Trap shift\nmethod", f=w1172) -> (s? t:f=w1170:dbl)
          n754 = Add(x=w1173, y=w1175) -> (x+y=w1176:dbl)
          n755 = Add(x=w1176, y=w1170) -> (x+y=w1232:dbl)
          n756 = Add(x=w1176, y=1.5707963267948966) -> (x+y=w1181:dbl)
          n757 = Add(x=w1232, y=1.5707963267948966) -> (x+y=w1245:dbl)
          n758 = Cosine(x=w1181) -> (cos(x)=w1259:dbl)
          n759 = Sine(x=w1181) -> (sin(x)=w1258:dbl)
          n760 = Multiply(x=w1259, y="Radius (MHz)") -> (x*y=w1252:dbl)
          n761 = Cosine(x=w1245) -> (cos(x)=w1257:dbl)
          n762 = Sine(x=w1245) -> (sin(x)=w1256:dbl)
          n763 = Multiply(x=w1258, y="Radius (MHz)") -> (x*y=w1251:dbl)
          n764 = Multiply(x=w1257, y="Radius (MHz)") -> (x*y=w1255:dbl)
          n765 = Multiply(x=w1256, y="Radius (MHz)") -> (x*y=w1253:dbl)
          n766 = Add(x=w1252, y=w1250) -> (x+y=w1201:dbl)
          n767 = Add(x=w1251, y=w1243) -> (x+y=w1199:dbl)
          n768 = Greater Or Equal?(x=w1184, y="N steps then stop") -> (x >= y?=w1242:bool)
          n769 = Add(x=w1255, y=w1254) -> (x+y=w1190:dbl)
          n770 = Add(x=w1253, y=w1243) -> (x+y=w1188:dbl)
          n771 = Not Equal To 0?(x="N steps then stop") -> (x != 0?=w1238:bool)
          n772 = And(x=w1242, y=w1238) -> (x .and. y?=w1239:bool)
          n773 = local read "Trap 1 sum mean"() -> (w1222:dbl)
          n774 = local read "Stop All"() -> (w1247:bool)
          n775 = local write "BD 1 Frequency 1 (MHz)"(w1201) -> ()
          n776 = local write "BD 2 Frequency 1 (MHz)"(w1199) -> ()
          n777 = local write "BD 1 Frequency 2 (MHz)"(w1190) -> ()
          n778 = local write "BD 2 Frequency 2 (MHz)"(w1188) -> ()
          n779 = Select(t=w1184, s="test", f=w1222) -> (s? t:f=→"Waveform Chart":dbl)
          n780 = Compound Arithmetic op=OR(w1247, "Stop Moving", w1239) -> (w1248:bool)
          n781 = local read "BD 1 Frequency 3 (MHz)"() -> (w1231:dbl)
          n782 = local read "BD 2 Frequency 3 (MHz)"() -> (w1230:dbl)
          n783 = Select(t=w1206, s="Reset graph", f=w1207) -> (s? t:f=w1187:dbl[])
          n784 = Select(t=w1206, s="Reset graph", f=w1208) -> (s? t:f=w1189:dbl[])
          n785 = Select(t=w1206, s="Reset graph", f=w1210) -> (s? t:f=w1198:dbl[])
          n786 = Select(t=w1206, s="Reset graph", f=w1211) -> (s? t:f=w1200:dbl[])
          n787 = Initialize Array(w1188, w1213) -> (w1214:dbl[])
          n788 = Initialize Array(w1199, w1213) -> (w1217:dbl[])
          n789 = Initialize Array(w1190, w1213) -> (w1215:dbl[])
          n790 = Initialize Array(w1201, w1213) -> (w1218:dbl[])
          n791 = local read "Y RF Frequency Limits (MHz)"() -> (w1228:T18)
          n792 = local read "X RF Frequency Limits (MHz)"() -> (w1229:T18)
          n793 = call "set RF board frequency - interlace.vi"("Board 2 Frequency Limits"=w1228, "Board 1 Frequency Limits"=w1229, "FPGA VI Reference In"=w1225, "Board 2 Frequency 3 (MHz)"=w1230, "Board 1 Frequency 3 (MHz)"=w1231, "Board 2 Frequency 2 (MHz)"=w1188, "Board 2 Frequency 1 (MHz)"=w1199, "Board 1 Frequency 2 (MHz)"=w1190, "Board 1 Frequency 1  (MHz)"=w1201) -> ()  [unwired: 1 in, 2 out]
          n794 = Bundle(w1215, w1214) -> (w1186:cluster{dbl[], dbl[]})  [unwired: 1 in]
          n795 = Bundle(w1218, w1217) -> (w1216:cluster{dbl[], dbl[]})  [unwired: 1 in]
          n796 = Build Array (concatenate)(w1201, w1200) -> (w1205:dbl[])
          n797 = Build Array (concatenate)(w1199, w1198) -> (w1203:dbl[])
          n798 = Build Array (concatenate)(w1190, w1189) -> (w1196:dbl[])
          n799 = Build Array (concatenate)(w1188, w1187) -> (w1194:dbl[])
          n800 = Bundle(w1205, w1203) -> (w1185:cluster{dbl[], dbl[]})  [unwired: 1 in]
          n801 = Bundle(w1196, w1194) -> (w1212:cluster{dbl[], dbl[]})  [unwired: 1 in]
          n802 = Build Array(w1216, w1186, w1185, w1212) -> (→"Trap trajectories":cluster{dbl[], dbl[]}[])
          n803 = case "To pause the process" shown="True" "Pause rotation" {
            frame False {
            }
            frame True {
              n804 = while {
                stop <- w1264 stop-if-true
                n805 = local read "Pause rotation"() -> (w1265:bool)
                n806 = Wait (ms)(milliseconds to wait=u32 10) -> ()  [unwired: 1 out]
                n807 = Not(x=w1265) -> (.not. x?=w1264:bool)
              }
            }
          }
          n808 = Decrement(x="N steps to plot") -> (x-1=w1191:i32)
          n809 = Array Subset(array=w1203, index=w1192, length=w1191) -> (w1202:dbl[])
          n810 = Array Subset(array=w1205, index=w1192, length=w1191) -> (w1204:dbl[])
          n811 = Array Subset(array=w1196, index=w1192, length=w1191) -> (w1195:dbl[])
          n812 = Array Subset(array=w1194, index=w1192, length=w1191) -> (w1193:dbl[])
          n813 = Quotient & Remainder(x=w1176, y=6.283185307179586) -> (x-y*floor(x/y)=w1177:dbl)  [unwired: 1 out]
          n814 = node-c288() -> ()  [unwired: 1 in, 1 out]
        }
        n815 = node-c288(w1157) -> ()  [unwired: 1 out]
        n816 = case shown="True" w1148 {
          tunnel: w1152 -> [_ w1163]
          tunnel: w1151 -> [_ w1162]
          tunnel: w1150 -> [_ w1161]
          tunnel: w1149 -> [_ w1160]
          frame False {
          }
          frame True {
            n817 = flat-sequence {
              tunnel: w1163 -> [w1167]
              tunnel: w1162 -> [w1166]
              tunnel: w1161 -> [w1165]
              tunnel: w1160 -> [w1164]
              frame #0 {
                n818 = local write "BD 1 Frequency 1 (MHz)"(w1167) -> ()
                n819 = local write "BD 2 Frequency 1 (MHz)"(w1166) -> ()
                n820 = local write "BD 1 Frequency 2 (MHz)"(w1165) -> ()
                n821 = local write "BD 2 Frequency 2 (MHz)"(w1164) -> ()
              }
              frame #1 {
                n822 = property on="Update all trap values" class="Bool (strict)"("Val(Sgnl)"=TRUE ("Value (Signaling)")) -> ()  [unwired: 2 in, 2 out]